vi "MartinsDCposition.vi"() -> ()   [LabVIEW 2011] (continued)
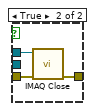
[diagram p3: hidden frame]
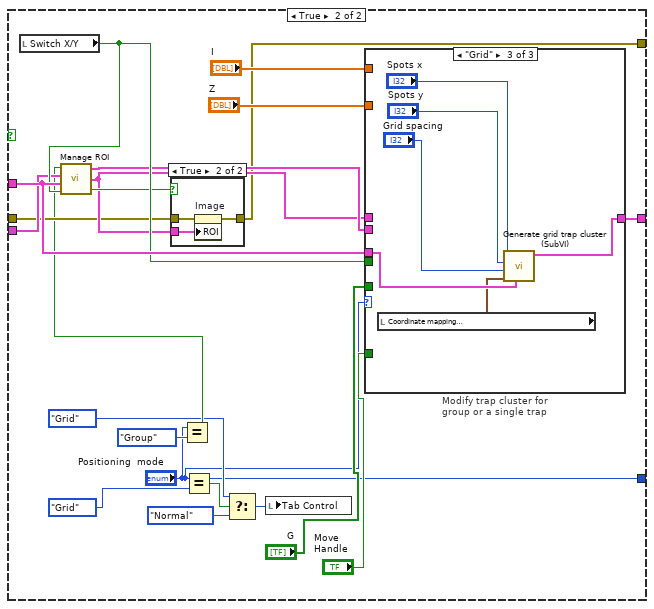
[diagram p8: hidden frame]
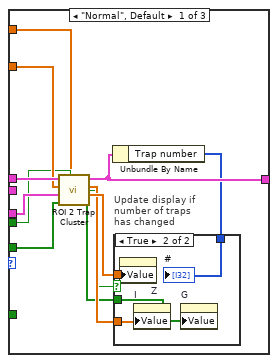
[diagram p10: hidden frame]
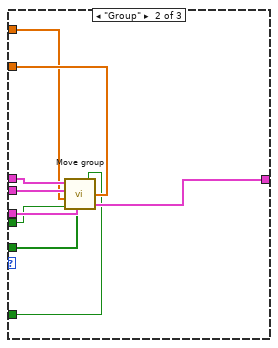
[diagram p12: hidden frame]
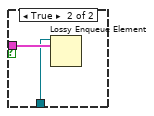
[diagram p14: hidden frame]
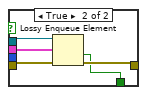
[diagram p16: hidden frame]
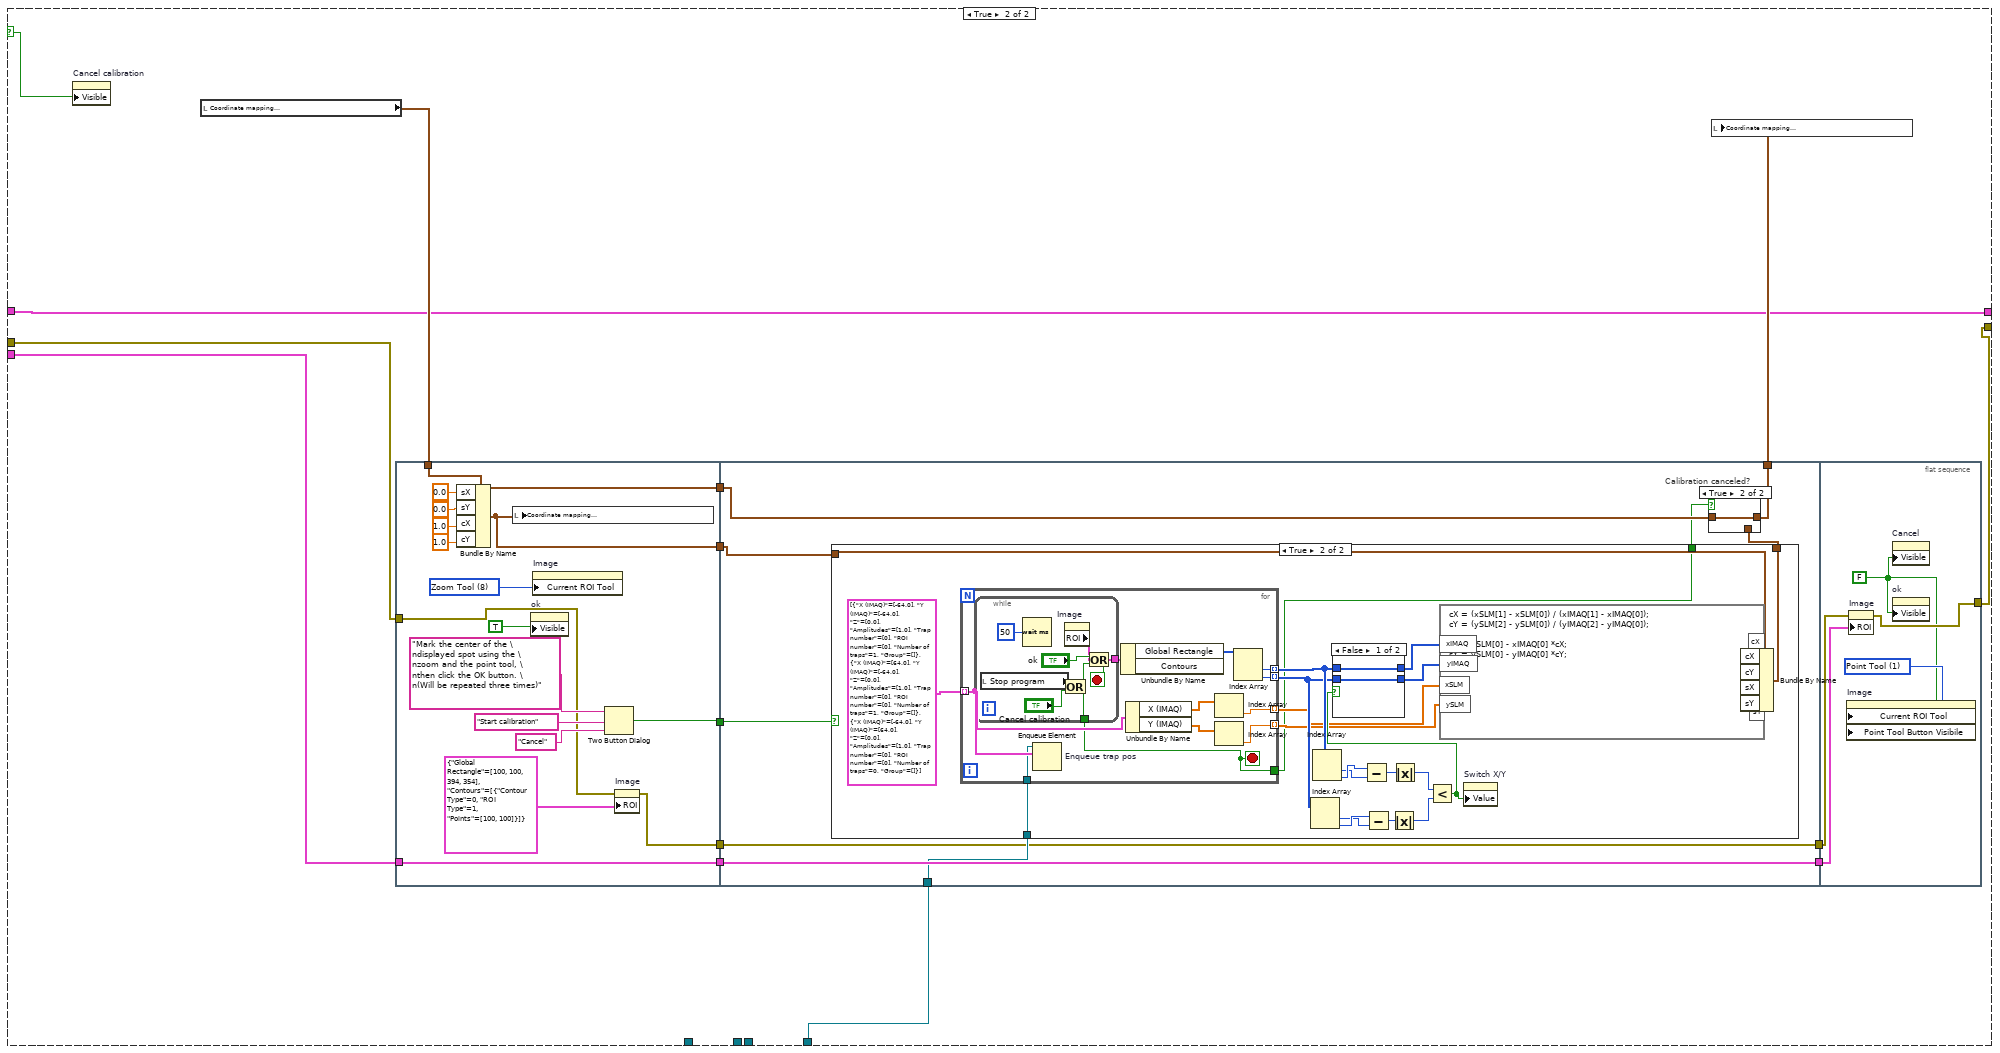
[diagram p20: hidden frame]
      }
      event "Create path": Value Change {
        n84 = event-data() -> ()  [unwired: 1 in, 5 out]
        n85 = property on="follow path" class="Bool (strict)"("Value"=FALSE) -> ()  [unwired: 2 in, 2 out]
        n86 = Flush Queue "Flush path \nwaypt queue"(queue=w215) -> ()  [unwired: 1 in, 3 out]
        n87 = Preview Queue Element(queue=w216) -> (element=w217:T3, error out=w220:errorcluster)  [unwired: 2 in, 2 out]
        n88 = Flush Queue "Flush path queue"(queue=w219) -> (queue out=w218:refnum<queue>)  [unwired: 1 in, 2 out]
        n89 = Enqueue Element "Enqueue current \ntrap pos in path"(queue=w218, element=w217) -> ()  [unwired: 2 in, 3 out]
        n90 = Enqueue Element "Enqueue current \ntrap pos in path \nwaypts"(queue=w215, element=w217, error in (no error)=w220) -> ()  [unwired: 1 in, 3 out]
      }
      event "cancel path": Value Change {
        n91 = event-data() -> ()  [unwired: 1 in, 5 out]
        n92 = local write "Create path"(FALSE ("Visible")) -> ()
      }
      event "Image", "Positioning  mode", "Z", "I", "Coordinate mapping \n(IMAQ to SLM)": Mouse Down; Key Up {
        n93 = event-data() -> ()  [unwired: 1 in, 3 out]
        n94 = local write "Updating trap cluster"(TRUE ("Update trap positions")) -> ()
      }
      event "Positioning  mode", "Z", "I", "Image", "Coordinate mapping \n(IMAQ to SLM)": Mouse Up {
        n95 = event-data() -> ()  [unwired: 1 in, 7 out]
        n96 = flat-sequence {
          frame #0 {
            n97 = Wait (ms)(milliseconds to wait=u32 100) -> ()  [unwired: 1 out]
          }
          frame #1 {
            n98 = local write "Updating trap cluster"(FALSE ("Update trap positions")) -> ()
          }
        }
      }
    }
    n99 = local read "Stop program"() -> (w197:bool)
  }
  n100 = while "Image acquisition loop" {
    tunnel: w4 -> [w238]
    tunnel: w6 -> [w254]
    tunnel: w8 -> [w253]
    tunnel: [w252] -> w53
    tunnel: [w234] -> w52
    tunnel: w51 -> [w248]
    tunnel: w49 -> [w240]
    shift-right: ["ROI size"] -> _
    shift-left: _ -> [_]
    tunnel: w46 -> [w239]
    tunnel: [w248] -> w44
    tunnel: [w235] -> w43
    tunnel: [w247] -> w42
    tunnel: w7 -> [w246]
    tunnel: w3 -> [w245]
    tunnel: w17 -> [w244]
    tunnel: w20 -> [w243]
    tunnel: w5 -> [w241]
    tunnel: w1 -> [w229]
    stop <- w251 stop-if-true
    n101 = Flush Queue(queue=w239) -> ()  [unwired: 1 in, 3 out]
    n102 = Flush Queue(queue=w240) -> ()  [unwired: 1 in, 3 out]
    n103 = Preview Queue Element(queue=w244, timeout in ms (-1)=10 ("f")) -> (element=w233:T3)  [unwired: 1 in, 3 out]
    n104 = Get Queue Status(queue=w243, return elements? (F)="Display path") -> (elements=w236:T3[])  [unwired: 1 in, 7 out]
    n105 = call <vilib>:"Acquire Semaphore.vi"("semaphore"=w229) -> ("semaphore out"=w231:T9)  [unwired: 4 in, 2 out]
    n106 = case shown="False" w238 {
      tunnel: w254 -> [w259 w271]
      tunnel: w253 -> [w258 w270]
      tunnel: [w258 w269] -> w252
      tunnel: [w257 w268] -> w234
      tunnel: [w259 w267] -> w235
      tunnel: [w260 w266] -> w247
      tunnel: w246 -> [w260 w265]
      tunnel: w245 -> [_ w264]
      tunnel: w241 -> [w257 w263]
      tunnel: [_ w262] -> _
      tunnel: w231 -> [w255 w261]
      tunnel: [w255 w261] -> w230
      frame False {
        n107 = Wait (ms)(milliseconds to wait=u32 100) -> ()  [unwired: 1 out]
      }
      frame True {
        n108 = case shown="False" w264 {
          tunnel: w271 -> [w279 w287]
          tunnel: [w277 w286] -> w269
          tunnel: [w276 w285] -> w268
          tunnel: w270 -> [w277 w284]
          tunnel: [w278 w283] -> w267
          tunnel: [w273 w282] -> w262
          tunnel: [w275 w281] -> w266
          tunnel: w265 -> [w274 w281]
          tunnel: w263 -> [w272 w280]
          frame False {
            n109 = call <vilib>:"IMAQdx Grab.vi"("error in"=w272, "Image In"=w279, "Session In"=w274) -> ("error out"=w276:errorcluster, "Buffer Number Out"=w273:u32, "Image Out"=w278:T2, "Session Out"=w275:T7)  [unwired: 5 in]
          }
          frame True {
            n110 = call <vilib>:"IMAQ Grab Acquire.vi"("error in (no error)"=w280, "Image In"=w287, "IMAQ Session In"=w284) -> ("error out"=w285:errorcluster, "Acquired Buffer Number"=w282:u32, "Image Out"=w283:T2, "IMAQ Session Out"=w286:refnum<k11>)  [unwired: 1 in, 4 out]
          }
        }
      }
    }
    n111 = call "Create trap overlay.vi"("Current trap cluster"=w233, "Image in"=w235, "ROI size"="ROI size", "Switch X/Y"="Switch X/Y", "Path"=w236) -> ()  [unwired: 1 out]
    n112 = case shown="True" "Show image" {
      tunnel: w235 -> [_ w288]
      frame False {
      }
      frame True {
        "Image" <- w288
      }
    }
    n113 = call <vilib>:"Release Semaphore.vi"("semaphore"=w230) -> ()  [unwired: 5 in, 2 out]
    n114 = local read "Stop program"() -> (w251:bool)
  }
  n115 = while "Trap position loop" {
    tunnel: w19 -> [w300]
    tunnel: w20 -> [w297]
    shift-right: [w299] -> _
    shift-left: w16 -> [w292]
    tunnel: w18 -> [w298]
    tunnel: w17 -> [w295]
    tunnel: [w294] -> w35
    tunnel: w21 -> [w291]
    tunnel: [w289] -> w33
    stop <- "Stop program" stop-if-true
    n116 = property on="Image" class="ImageControl"(error in=w291) -> (error out=w290:errorcluster, "ROI"=w294:T1)  [unwired: 1 in, 1 out]
    n117 = case shown="False" "Run calibration" {
      selector: "Run calibration" -> [_ w494]
      tunnel: w300 -> [w325 _]
      tunnel: w292 -> [w324 w493]
      tunnel: [w304 w493] -> w299
      tunnel: w298 -> [w315 w503]
      tunnel: w297 -> [w313 _]
      tunnel: w295 -> [w310 _]
      tunnel: w294 -> [w309 w502]
      tunnel: w290 -> [w308 w498]
      tunnel: [w306 w495] -> w289
      frame False {
        n118 = case "Update trap cluster" shown="False" "Updating trap cluster" {
          tunnel: w324 -> [w327 w348]
          tunnel: [w327 w341] -> w316
          tunnel: w309 -> [_ w339]
          tunnel: w308 -> [w326 w338]
          tunnel: [w326 w337] -> w307
          tunnel: [_ "Positioning  mode"] -> w301
          frame False {
          }
          frame True {
            n119 = local read "Switch X/Y"() -> (w347:bool)
            n120 = Equal?(x="Positioning  mode", y=enum16{"Normal", "Group", "Grid"}."Group") -> (x = y?=w335:bool)
            n121 = call "Manage ROI.vi"("Switch X/Y"=w347, "Trap cluster in"=w348, "ROI in"=w339, "Group traps"=w335) -> ("Replace ROI"=w346:bool, "ROI out"=w340:T1, "Previous ROI out"=w345:T1)
            n122 = case shown="True" w346 {
              tunnel: w340 -> [_ w352]
              tunnel: w338 -> [w349 w351]
              tunnel: [w349 w350] -> w337
              frame False {
              }
              frame True {
                n123 = property on="Image" class="ImageControl"(error in=w351, "ROI"=w352) -> (error out=w350:errorcluster)  [unwired: 1 in, 1 out]
              }
            }
            n124 = Equal?(x="Positioning  mode", y=enum16{"Normal", "Group", "Grid"}."Grid") -> (x = y?=w333:bool)
            n125 = Select(t=enum32{"Normal", "Grid"}."Grid", s=w333, f=enum32{"Normal", "Grid"}."Normal" ("Tab Control")) -> (s? t:f=w330:enum32{"Normal", "Grid"})
            n126 = local write "Tab Control"(w330) -> ()
            n127 = case "Modify trap cluster for \ngroup or a single trap" shown="\"Grid\"" "Positioning  mode" {
              tunnel: [w357 w374 w379] -> w341
              tunnel: w340 -> [w364 w375 _]
              tunnel: w348 -> [w363 w377 w380]
              tunnel: w345 -> [_ w376 _]
              tunnel: "Z" -> [w362 w373 _]
              tunnel: "Move \nHandle" -> [_ w372 _]
              tunnel: w347 -> [w361 w371 _]
              tunnel: "I" -> [w359 w370 _]
              tunnel: "G" -> [w354 w369 _]
              frame "Normal", Default {
                n128 = call "ROI 2 Trap Cluster.vi"("Amplitudes"=w359, "Switch X/Y"=w361, "Group"=w354, "Trap Cluster in"=w363, "Z"=w362, "ROI"=w364) -> ("Group out"=w353:bool[], "Z out"=w360:dbl[], "Amplitudes out"=w358:dbl[], "Trap Cluster Out"=w357:T3, "Update display"=w355:bool)
                n129 = Unbundle By Name(w357) -> ("Trap number"=w356:i32[])
                n130 = case "Update display if\nnumber of traps \nhas changed" shown="True" w355 {
                  tunnel: w360 -> [_ w368]
                  tunnel: w358 -> [_ w367]
                  tunnel: w356 -> [_ w366]
                  tunnel: w353 -> [_ w365]
                  frame False {
                  }
                  frame True {
                    n131 = property on="Z" class="Arr (strict)"("Value"=w368) -> ()  [unwired: 2 in, 2 out]
                    n132 = property on="I" class="Arr (strict)"("Value"=w367) -> ()  [unwired: 2 in, 2 out]
                    n133 = property on="G" class="Arr (strict)"("Value"=w365) -> ()  [unwired: 2 in, 2 out]
                    "#" <- w366
                  }
                }
              }
              frame "Group" {
                n134 = call "Move group.vi"("New handle position in"=w375, "Trap cluster in"=w377, "Previous handle position in"=w376, "Amplitudes"=w370, "Group"=w369, "Switch X/Y"=w371, "Move handle"=w372, "Z"=w373) -> ("Trap cluster out"=w374:T3)
              }
              frame "Grid" {
                n135 = local read "Coordinate mapping \n(IMAQ to SLM)"() -> (w378:T5)
                n136 = call "Generate grid trap cluster (SubVI).vi"("output cluster 3"=w380, "Coordinate mapping \n(IMAQ to SLM)"=w378, "Grid spacing"="Grid spacing", "Spots y"="Spots y", "Spots x"="Spots x") -> ("output cluster 2"=w379:T3)  [unwired: 6 in]
              }
            }
          }
        }
        n137 = Wait (ms)(milliseconds to wait=u32 50) -> ()  [unwired: 1 out]
        n138 = Unbundle By Name("Path controls") -> ("Add current \npositions to path"=w311:bool, "Synchronize traps"=w320:bool, "Step length"=w302:dbl, "follow path"=w314:bool, "Arrive \nsimultaneously"=w322:bool)
        n139 = Or(x=w311, y=w320) -> (x .or. y?=w321:bool)
        n140 = Or(x=w320, y=w314) -> (x .or. y?=w318:bool)
        n141 = Or(x=w321, y=w314) -> (x .or. y?=w319:bool)
        n142 = case shown="True" "Create path" {
          tunnel: w325 -> [_ w398]
          tunnel: w316 -> [w384 w392]
          tunnel: w302 -> [_ w406]
          tunnel: w313 -> [_ w402]
          tunnel: w322 -> [_ w405]
          tunnel: w319 -> [_ w404]
          tunnel: w318 -> [_ w403]
          tunnel: w314 -> [_ w391]
          tunnel: w315 -> [w387 w399]
          tunnel: w310 -> [_ w397]
          tunnel: w309 -> [_ w396]
          tunnel: w307 -> [w386 w395]
          tunnel: [w386 w394] -> w306
          tunnel: "Updating trap cluster" -> [w385 _]
          tunnel: [w384 w393] -> w304
          tunnel: w301 -> [_ w390]
          frame False {
            n143 = case shown="False" w385 {
              tunnel: w384 -> [_ w389]
              tunnel: w387 -> [_ w388]
              frame False {
              }
              frame True {
                n144 = Lossy Enqueue Element(queue=w388, element=w389) -> ()  [unwired: 1 in, 4 out]
              }
            }
          }
          frame True {
            n145 = Lossy Enqueue Element "Enqueue\noverlay pos"(queue=w397, element=w392) -> ()  [unwired: 1 in, 4 out]
            n146 = case "Add wpt" shown="True" w404 {
              tunnel: w392 -> [_ w484]
              tunnel: w398 -> [w481 w485]
              tunnel: [w481 w482] -> w407
              tunnel: [_ w483] -> w400
              frame False {
              }
              frame True {
                n147 = Enqueue Element "Enqueue path\n waypts"(queue=w485, element=w484) -> (queue out=w482:refnum<queue>, error out=w483:errorcluster)  [unwired: 2 in, 1 out]
              }
            }
            n148 = case "Compute path" shown="True" w403 {
              tunnel: w407 -> [_ w492]
              tunnel: w402 -> [_ w491]
              tunnel: w406 -> [_ w490]
              tunnel: w405 -> [_ w489]
              tunnel: [w486 w487] -> w401
              tunnel: w400 -> [w486 w488]
              frame False {
              }
              frame True {
                n149 = call "compute path cluster.vi"("path queue"=w491, "Arrive simultaeously"=w489, "error in (no error)"=w488, "Step length\n(IMAQ pixels)"=w490, "waypoint queue"=w492) -> ("error out"=w487:errorcluster)  [unwired: 2 in]
              }
            }
            n150 = case "Follow path" shown="True" w391 {
              tunnel: w402 -> [_ w437]
              tunnel: w401 -> [_ w438]
              tunnel: w399 -> [_ w440]
              tunnel: w398 -> [_ w439]
              tunnel: w396 -> [_ w436]
              tunnel: w395 -> [w409 w417]
              tunnel: [w409 w416] -> w394
              tunnel: [w408 w411] -> w393
              tunnel: w392 -> [w408 _]
              tunnel: w390 -> [_ w410]
              frame False {
              }
              frame True {
                w431 = TRUE ("Visible")
                n151 = Flush Queue "Flush Waypts"(queue=w439, error in (no error)=w438) -> (error out=w430:errorcluster)  [unwired: 2 out]
                n152 = Get Queue Status(queue=w437, error in (no error)=w430) -> (queue out=w434:refnum<queue>, error out=w429:errorcluster, # elements in queue=w433:i32)  [unwired: 1 in, 5 out]
                n153 = property on="Pause" class="Bool (strict)"(error in=w429, "Visible"=w431) -> (error out=w428:errorcluster)  [unwired: 1 in, 1 out]
                n154 = property on="cancel path" class="Bool"(error in=w428, "Visible"=w431) -> (error out=w427:errorcluster)  [unwired: 1 in, 1 out]
                n155 = for {
                  N: w433 -> [_]
                  tunnel: w427 -> [w459]
                  tunnel: w440 -> [w461]
                  tunnel: w434 -> [w457]
                  tunnel: [w457] -> w432
                  tunnel: [FALSE ("Group traps")] -> w412
                  shift-right: [w448] -> w411
                  shift-left: _ -> [w450]
                  tunnel: [w447] -> w426
                  tunnel: [w444] -> w424 mode=indexing
                  tunnel: [w445] -> w420
                  tunnel: [TRUE ("Display path")] -> w418
                  tunnel: w410 -> [_]
                  i -> [w445]
                  stop <- w454 stop-if-true
                  n156 = Dequeue Element(queue=w457, timeout in ms (-1)=0, error in (no error)=w459) -> (element=w449:T3, timed out?=w453:bool, error out=w460:errorcluster)  [unwired: 1 out]
                  n157 = while {
                    tunnel: [w478] -> w451
                    tunnel: ["cancel path"] -> w446
                    stop <- w480 stop-if-true
                    n158 = local read "Stop program"() -> (w478:bool)
                    n159 = Wait (ms)(milliseconds to wait="Step time \n(ms)") -> ()  [unwired: 1 out]
                    n160 = Or(x=w478, y="cancel path") -> (x .or. y?=w476:bool)
                    n161 = Implies(1:w476, 2:"Pause") -> (0:w480:bool)
                  }
                  n162 = case shown="False" "Skip step if \ntimed out" {
                    tunnel: w461 -> [w467 w472]
                    tunnel: w460 -> [w466 w470]
                    tunnel: [FALSE ("overflow?") w468] -> w452
                    tunnel: w449 -> [w465 w471]
                    tunnel: [w464 w469] -> w447
                    tunnel: 2000 ("timeout in ms (-1)") -> [w463 _]
                    frame False {
                      n163 = Enqueue Element "Enqueue trap pos"(queue=w467, element=w465, timeout in ms (-1)=w463, error in (no error)=w466) -> (error out=w464:errorcluster)  [unwired: 2 out]
                    }
                    frame True {
                      n164 = Lossy Enqueue Element(queue=w472, element=w471, error in (no error)=w470) -> (overflow?=w468:bool, error out=w469:errorcluster)  [unwired: 2 out]
                    }
                  }
                  "Step skipped" <- w452
                  n165 = case shown="False" w451 {
                    tunnel: w450 -> [_ w474]
                    tunnel: w449 -> [w473 _]
                    tunnel: [w473 w474] -> w448
                    frame False {
                    }
                    frame True {
                    }
                  }
                  n166 = Or(x=w446, y=w451) -> (x .or. y?=w456:bool)
                  n167 = Or(x=w456, y=w453) -> (x .or. y?=w454:bool)
                  n168 = Tick Count (ms)() -> (millisecond timer value=w444:u32)
                }
                n169 = local write "Display path"(FALSE ("Display path")) -> ()
                n170 = local read "Switch X/Y"() -> (w414:bool)
                n171 = call "Trap cluster 2 ROI.vi"("Switch X/Y"=w414, "Trap cluster"=w411, "ROI in"=w436) -> ("ROI out"=w435:T1)
                n172 = local write "Positioning  mode"(w410) -> ()
                n173 = local write "Step skipped"(w412) -> ()
                n174 = local write "Display path"(w418) -> ()
                n175 = local write "Create path"(w412) -> ()
                n176 = property on="Pause" class="Bool (strict)"(error in=w426, "Visible"=w412, "Value"=w412) -> (error out=w425:errorcluster)  [unwired: 1 in, 1 out]
                n177 = property on="cancel path" class="Bool"(error in=w425, "Visible"=w412) -> ()  [unwired: 1 in, 2 out]
                n178 = property on="Image" class="ImageControl"(error in=w417, "ROI"=w435) -> (error out=w416:errorcluster)  [unwired: 1 in, 1 out]
                n179 = property on="follow path" class="Bool (strict)"("Value"=w412) -> ()  [unwired: 2 in, 2 out]
                n180 = Array Max & Min(array=w424) -> (max value=w423:u32, min value=w422:u32)  [unwired: 2 out]
                n181 = Subtract(x=w423, y=w422) -> (x-y=w421:u32)
                n182 = Increment(x=w420) -> (x+1=w415:i32)
                n183 = Divide(x=w421, y=w415) -> (x/y=→"Average step time (ms)":dbl)
                n184 = Flush Queue "Flush Path"(queue=w432) -> ()  [unwired: 1 in, 3 out]
              }
            }
          }
        }
        n185 = case shown="True" "Apply Corrections" {
          frame False {
          }
          frame True {
            n186 = call "Apply Corrections.vi"() -> ()  [unwired: 1 in]
          }
        }
      }
      frame True {
        n187 = property on="Cancel calibration" class="Bool"("Visible"=w494) -> ()  [unwired: 2 in, 2 out]
        n188 = local read "Coordinate mapping \n(IMAQ to SLM)"() -> (w501:T5)
        n189 = flat-sequence {
          tunnel: [w517] -> w507
          tunnel: [w519] -> w506
          tunnel: w502 -> [w517]
          tunnel: w501 -> [w511]
          tunnel: [w508] -> w500
          tunnel: [w511] -> w499
          tunnel: w498 -> [w510]
          tunnel: [w509] -> w496
          tunnel: [w532] -> w505
          tunnel: w507 -> [w532]
          tunnel: w506 -> [w526]
          tunnel: [w528] -> w504
          tunnel: w503 -> [w531]
          tunnel: w500 -> [w530]
          tunnel: w499 -> [w527]
          tunnel: [w524] -> w497
          tunnel: w496 -> [w524]
          tunnel: w505 -> [w587]
          tunnel: w497 -> [w585]
          tunnel: [w584] -> w495
          frame #0 {
            w520 = u32 8 items=["Zoom Tool"=8, "Selection Tool"=0, "Pan Tool"=9, "Point Tool"=1, "Line Tool"=2, "Rectangle Tool"=3, "Rotated Rectangle Tool"=12, "Polyline Tool"=10, "Polygon Tool"=5, "Freehand Tool"=11, "Closed Freehand Tool"=6, "Ellipse Tool"=4, "Annulus Tool"=7] ("Current ROI Tool")
            n190 = Bundle By Name(cluster=w511, "sX"=0.0, "sY"=0.0, "cX"=1.0 ("sX"), "cY"=1.0) -> (w508:T5)
            n191 = local write "Coordinate mapping \n(IMAQ to SLM)"(w508) -> ()
            n192 = property on="ok" class="Bool"("Visible"=TRUE ("ROI Tool Buttons Visibile:Zoom Tool Button Visible")) -> ()  [unwired: 2 in, 2 out]
            n193 = property on="Image" class="ImageControl"("Current ROI Tool"=w520) -> ()  [unwired: 2 in, 2 out]
            n194 = Two Button Dialog(message="Mark the center of the \ndisplayed spot using the \nzoom and the point tool, \nthen click the OK button. \n(Will be repeated three times)", 1:"Cancel" ("F button name (\"Cancel\")"), 2:"Start calibration" ("T button name (\"OK\")")) -> (T button?=w519:bool)
            n195 = property on="Image" class="ImageControl"(error in=w510, "ROI"=T1 {"Global Rectangle"=[100, 100, 394, 354], "Contours"=[{"Contour Type"=0, "ROI Type"=1, "Points"=[100, 100]}]} ("ROI 2")) -> (error out=w509:errorcluster)  [unwired: 1 in, 1 out]
          }
          frame #1 {
            n196 = case shown="True" w526 {
              tunnel: w530 -> [w536 w547]
              tunnel: [w536 w542] -> w529
              tunnel: w531 -> [_ w538]
              tunnel: [TRUE ("Stop program") w537] -> w525
              frame False {
              }
              frame True {
                n197 = for {
                  tunnel: [w574] -> w556 mode=indexing
                  tunnel: [w573] -> w555 mode=indexing
                  tunnel: T3[] [{"X (IMAQ)"=[-64.0], "Y (IMAQ)"=[-64.0], "Z"=[0.0], "Amplitudes"=[1.0], "Trap number"=[0], "ROI number"=[0], "Number of traps"=1, "Group"=[]}, {"X (IMAQ)"=[64.0], "Y (IMAQ)"=[-64.0], "Z"=[0.0], "Amplitudes"=[1.0], "Trap number"=[0], "ROI number"=[0], "Number of traps"=1, "Group"=[]}, {"X (IMAQ)"=[-64.0], "Y (IMAQ)"=[64.0], "Z"=[0.0], "Amplitudes"=[1.0], "Trap number"=[0], "ROI number"=[0], "Number of traps"=0, "Group"=[]}] -> [w571] mode=indexing
                  tunnel: [w568] -> w540 mode=indexing
                  tunnel: [w566] -> w539 mode=indexing
                  tunnel: w538 -> [w570]
                  tunnel: [w565] -> w537
                  stop <- w565 stop-if-true
                  n198 = while {
                    tunnel: [w581] -> w572
                    tunnel: [w577] -> w565
                    stop <- w579 stop-if-true
                    n199 = local read "Stop program"() -> (w578:bool)
                    n200 = Wait (ms)(milliseconds to wait=u32 50) -> ()  [unwired: 1 out]
                    n201 = Or(x=w578, y="Cancel calibration") -> (x .or. y?=w577:bool)
                    n202 = property on="Image" class="ImageControl"() -> ("ROI"=w581:T1)  [unwired: 2 in, 2 out]
                    n203 = Or(x="ok", y=w577) -> (x .or. y?=w579:bool)
                  }
                  n204 = Enqueue Element "Enqueue trap pos"(queue=w570, element=w571) -> ()  [unwired: 2 in, 3 out]
                  n205 = Unbundle By Name(w572) -> ("Global Rectangle"=w575:i32[])  [unwired: 1 out]
                  n206 = Unbundle By Name(w571) -> ("X (IMAQ)"=w569:dbl[], "Y (IMAQ)"=w567:dbl[])
                  n207 = Index Array(array=w569) -> (element=w568:dbl)  [unwired: 1 in]
                  n208 = Index Array(array=w567) -> (element=w566:dbl)  [unwired: 1 in]
                  n209 = Index Array(array=w575) -> (element #1=w574:i32, element #2=w573:i32)  [unwired: 2 in]
                }
                n210 = Index Array(array=w555) -> (element #1=w557:i32, element #2=w558:i32)  [unwired: 2 in]
                n211 = Index Array(array=w556) -> (element #1=w559:i32, element #2=w560:i32)  [unwired: 2 in]
                n212 = Subtract(x=w560, y=w559) -> (x-y=w552:i32)
                n213 = Subtract(x=w558, y=w557) -> (x-y=w550:i32)
                n214 = Absolute Value(x=w550) -> (abs(x)=w549:i32)
                n215 = Absolute Value(x=w552) -> (abs(x)=w551:i32)
                n216 = Less?(x=w551, y=w549) -> (x < y?=w548:bool)
                n217 = case shown="False" w548 {
                  tunnel: w556 -> [w562 w564]
                  tunnel: w555 -> [w561 w563]
                  tunnel: [w561 w564] -> w553
                  tunnel: [w562 w563] -> w554
                  frame False {
                  }
                  frame True {
                  }
                }
                n218 = formula code="cX = (xSLM[1] - xSLM[0]) / (xIMAQ[1] - xIMAQ[0]); \ncY = (ySLM[2] - ySLM[0]) / (yIMAQ[2] - yIMAQ[0]); \n\nsX = xSLM[0] - xIMAQ[0] *cX;\nsY = ySLM[0] - yIMAQ[0] *cY;"("xIMAQ"=w554, "yIMAQ"=w553, "xSLM"=w540, "ySLM"=w539) -> ("cX"=w546:dbl, "cY"=w545:dbl, "sX"=w544:dbl, "sY"=w543:dbl)
                n219 = property on="Switch X/Y" class="Bool (strict)"("Value"=w548) -> ()  [unwired: 2 in, 2 out]
                n220 = Bundle By Name(cluster=w547, "cX"=w546, "cY"=w545, "sX"=w544, "sY"=w543) -> (w542:T5)
              }
            }
            n221 = case "Calibration canceled?" shown="True" w525 {
              tunnel: w529 -> [w533 _]
              tunnel: [w533 w534] -> w528
              tunnel: w527 -> [_ w534]
              frame False {
              }
              frame True {
              }
            }
          }
          frame #2 {
            w583 = FALSE ("ROI Tool Buttons Visibile:Zoom Tool Button Visible")
            w586 = u32 1 items=["Zoom Tool"=8, "Selection Tool"=0, "Pan Tool"=9, "Point Tool"=1, "Line Tool"=2, "Rectangle Tool"=3, "Rotated Rectangle Tool"=12, "Polyline Tool"=10, "Polygon Tool"=5, "Freehand Tool"=11, "Closed Freehand Tool"=6, "Ellipse Tool"=4, "Annulus Tool"=7] ("Current ROI Tool")
            n222 = property on="Image" class="ImageControl"("Current ROI Tool"=w586, "Point Tool Button Visibile"=w583) -> ()  [unwired: 2 in, 2 out]
            n223 = property on="Image" class="ImageControl"(error in=w585, "ROI"=w587) -> (error out=w584:errorcluster)  [unwired: 1 in, 1 out]
            n224 = property on="Cancel" class="Bool"("Visible"=w583) -> ()  [unwired: 2 in, 2 out]
            n225 = property on="ok" class="Bool"("Visible"=w583) -> ()  [unwired: 2 in, 2 out]
          }
        }
        n226 = local write "Coordinate mapping \n(IMAQ to SLM)"(w504) -> ()
      }
    }
  }
  n227 = property on="Show image" class="Bool (strict)"("Visible"=w41) -> ()  [unwired: 2 in, 2 out]
  n228 = property on="ROI size" class="DigNum (strict)"("Visible"=w41) -> ()  [unwired: 2 in, 2 out]
  n229 = property on="Measure" class="Bool"("Visible"=w41) -> ()  [unwired: 2 in, 2 out]
  n230 = call-poly <vilib>:"Close Input Device.vi"("error in (no error)"=w27, "device ID"=w29) -> ()  [unwired: 9 out]
  n231 = call "FreeGPUandSLM.vi"("error in"=w32) -> ("error out"=w31:errorcluster)  [unwired: 1 out]
  "CUDA/SLM error" <- w31
  n232 = case shown="True" w4 {
    tunnel: w53 -> [_ w593]
    tunnel: w52 -> [w588 w592]
    tunnel: w42 -> [_ w591]
    tunnel: w3 -> [_ w590]
    tunnel: [w588 w589] -> w34
    frame False {
    }
    frame True {
      n233 = case shown="False" w590 {
        tunnel: w593 -> [_ w599]
        tunnel: w592 -> [w596 w598]
        tunnel: [w595 w597] -> w589
        tunnel: w591 -> [w594 _]
        frame False {
          n234 = call <vilib>:"IMAQdx Close Camera.vi"("error in"=w596, "Session In"=w594) -> ("error out"=w595:errorcluster)  [unwired: 9 in]
        }
        frame True {
          n235 = call <vilib>:"IMAQ Close.vi"("error in (no error)"=w598, "IMAQ Session In"=w599) -> ("error out"=w597:errorcluster)  [unwired: 9 in]
        }
      }
    }
  }
  n236 = Merge Errors(w34, w33) -> (w30:errorcluster)
  "NI Vision error" <- w30
  n237 = call "IMAQ Dispose"("Image"=w43) -> ()  [unwired: 5 in, 1 out]
  n238 = for {
    tunnel: w44 -> [w600] mode=indexing
    n239 = call "IMAQ Dispose"("Image"=w600) -> ()  [unwired: 5 in, 1 out]
  }
  n240 = Unbundle By Name(w35) -> ("Contours"=w40:T12)
  n241 = Index Array(array=w40) -> (element=w39:T13)  [unwired: 1 in]
  n242 = flat-sequence {
    tunnel: w31 -> [_]
    tunnel: w30 -> [_]
    frame #0 {
      n243 = local write "Stop program"(FALSE ("Stop program")) -> ()
    }
  }
  n244 = Unbundle By Name(w39) -> ("ROI Type"=w38:u32)
  n245 = Equal?(x=w38, y=u32 1) -> (x = y?=w36:bool)
  n246 = case shown="True" w36 {
    tunnel: w35 -> [_ w602]
    frame False {
    }
    frame True {
      n247 = local write "ROI"(w602) -> ()
    }
  }
